vi "front_panel_v2.vi"() -> ()   [LabVIEW 2021]
uses:
  <vilib>/Platform/TimedLoop/XDataNode/timing_clust.ctl
  <vilib>/Platform/TimedLoop/XDataNode/nitl_modes.ctl
  <vilib>/Platform/TimedLoop/XDataNode/wakeup.ctl
  Global 1.vi
  <vilib>/platform/TimedLoop/XDataNode/XDataNode.xnode
  <vilib>/Platform/TimedLoop/XDataNode/XDNodeRunTimeDep.lvlib
panel:
  in  "Glove Address":string
  in  "Robotic Hand Address":string="192.168.4.93"
  out "Thumb 3":dbl
  out "Index Finger 2":dbl
  out "Middle Finger3":dbl
  out "Ring Finger 3":dbl
  out "Pinky Finger 2":dbl
  out "Simulation Connected":bool
  in  "Stop":bool
  out "Hand Status":bool
  out "Glove Status":bool
  in  "Stop Execution":bool
  in  "?":enum32{"Imitation", "Manual Control"}(tab)=enum."Manual Control"
  out "Glove Signal":dbl[](array[numeric])
  in  "Stop Imitation":bool
  out "Finger Positions From Glove":dbl[](graph)
  out "Finger Positions":T1(graph)
  in  "Stop Manual Control":bool
  out "Output From Knob":string
  in  "Pinky":dbl(slide) scale=0.0..-47.0
  in  "Ring Finger":dbl(slide) scale=0.0..-60.0
  in  "Index":dbl(slide) scale=0.0..-20.0
  in  "Middle Finger":dbl(slide)=85.0 scale=85.0..4.0
  in  "Thumb":dbl(slide)=90.0
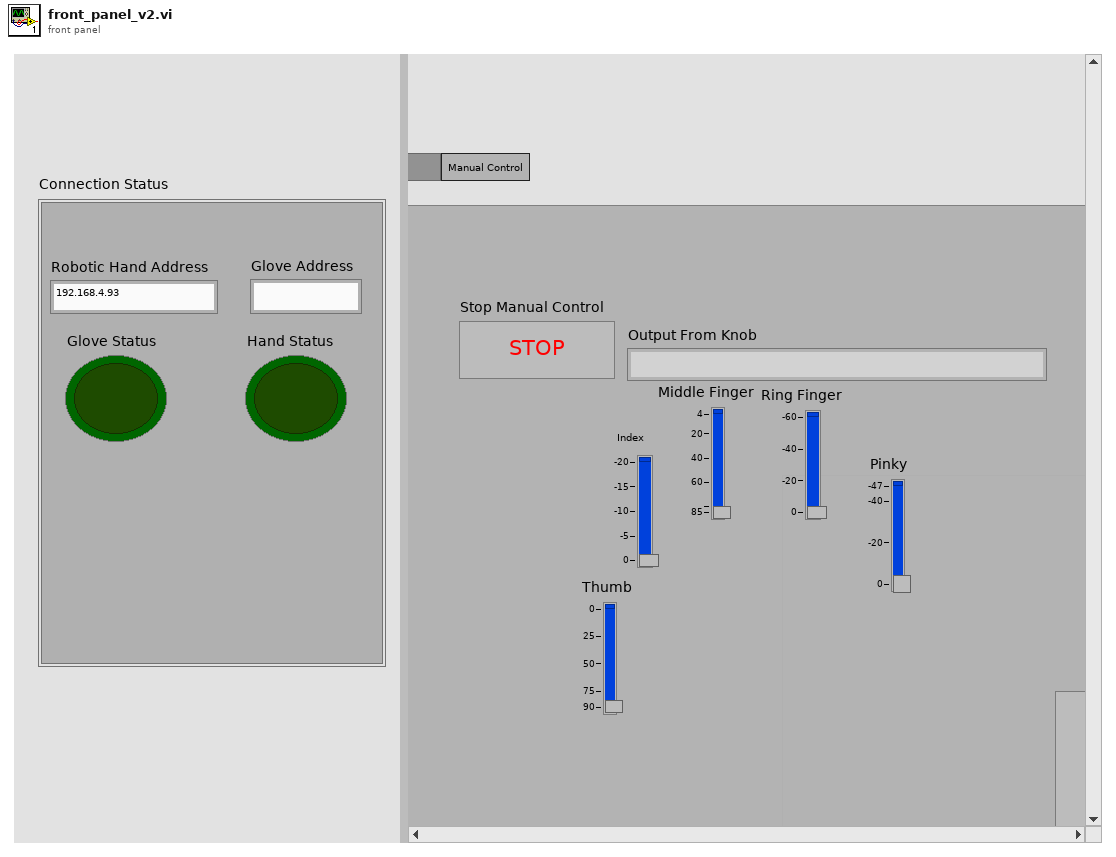
[diagram p1: front panel]
types:
  T1 = cluster{"[0]":dbl, "[1]":dbl, "[2]":dbl, "[3]":dbl, "[4]":dbl, "[5]":dbl, "[6]":dbl, "[7]":dbl, "[8]":dbl}
  T2 = cluster{"Clients":refnum<k5>[], "Listener":refnum<k5>}
  T3 = enum16{"Initialize", "Status Check", "Send Data", "Stop"}
  T4 = enum16{"Standard", "Buffered", "CRLF", "Immediate"}
  T5 = typedef "XDNodeRunTimeDep.lvlib/timing_clust.ctl" = cluster{"Expected End [f-1]":u64, "Actual End [f-1]":u64, "Finished Late? [f-1]":bool, "Expected End [i-1]":u64, "Actual End [i-1]":u64, "Finished Late? [i-1]":bool, "Expected Start [i]":u64, "Actual Start [i]":u64, "Expected Start [f]":u64, "Actual Start [f]":u64, "Source Name":string, "Structure Name":string, "Period":i64, "Deadline":i64, "Offset":i64, "Start":i64, "Priority":i32, "Timeout":i32, "Mode":T6, "Wakeup Reason":T7, "Error":errorcluster, "Source Type":string, "Secondary Source Type":string, "Global End Time":u64, "Global Start Time":u64, "Frame Duration":u64, "Iteration Duration":u64, "Assigned CPU":i32, "I/O Scan Engine Mode":u32}
  T6 = typedef "XDNodeRunTimeDep.lvlib/nitl_modes.ctl" = enum32{"No Change", "Process missed periods, maintain original phase", "Discard missed periods, maintain original phase", "Process missed periods, ignore original phase", "Discard missed periods, ignore original phase"}
  T7 = typedef "XDNodeRunTimeDep.lvlib/wakeup.ctl" = enum32{"Normal", "Aborted", "Asynchronous wakeup", "Timing source error", "Timed loop error", "Timeout"}
  T8 = cluster{"Glove output RT[0]":dbl, "Glove output RT[1]":dbl, "Glove output RT[2]":dbl, "Glove output RT[3]":dbl, "Glove output RT[4]":dbl, "Glove output RT[5]":dbl, "Glove output RT[6]":dbl, "Glove output RT[7]":dbl, "Glove output RT[8]":dbl}
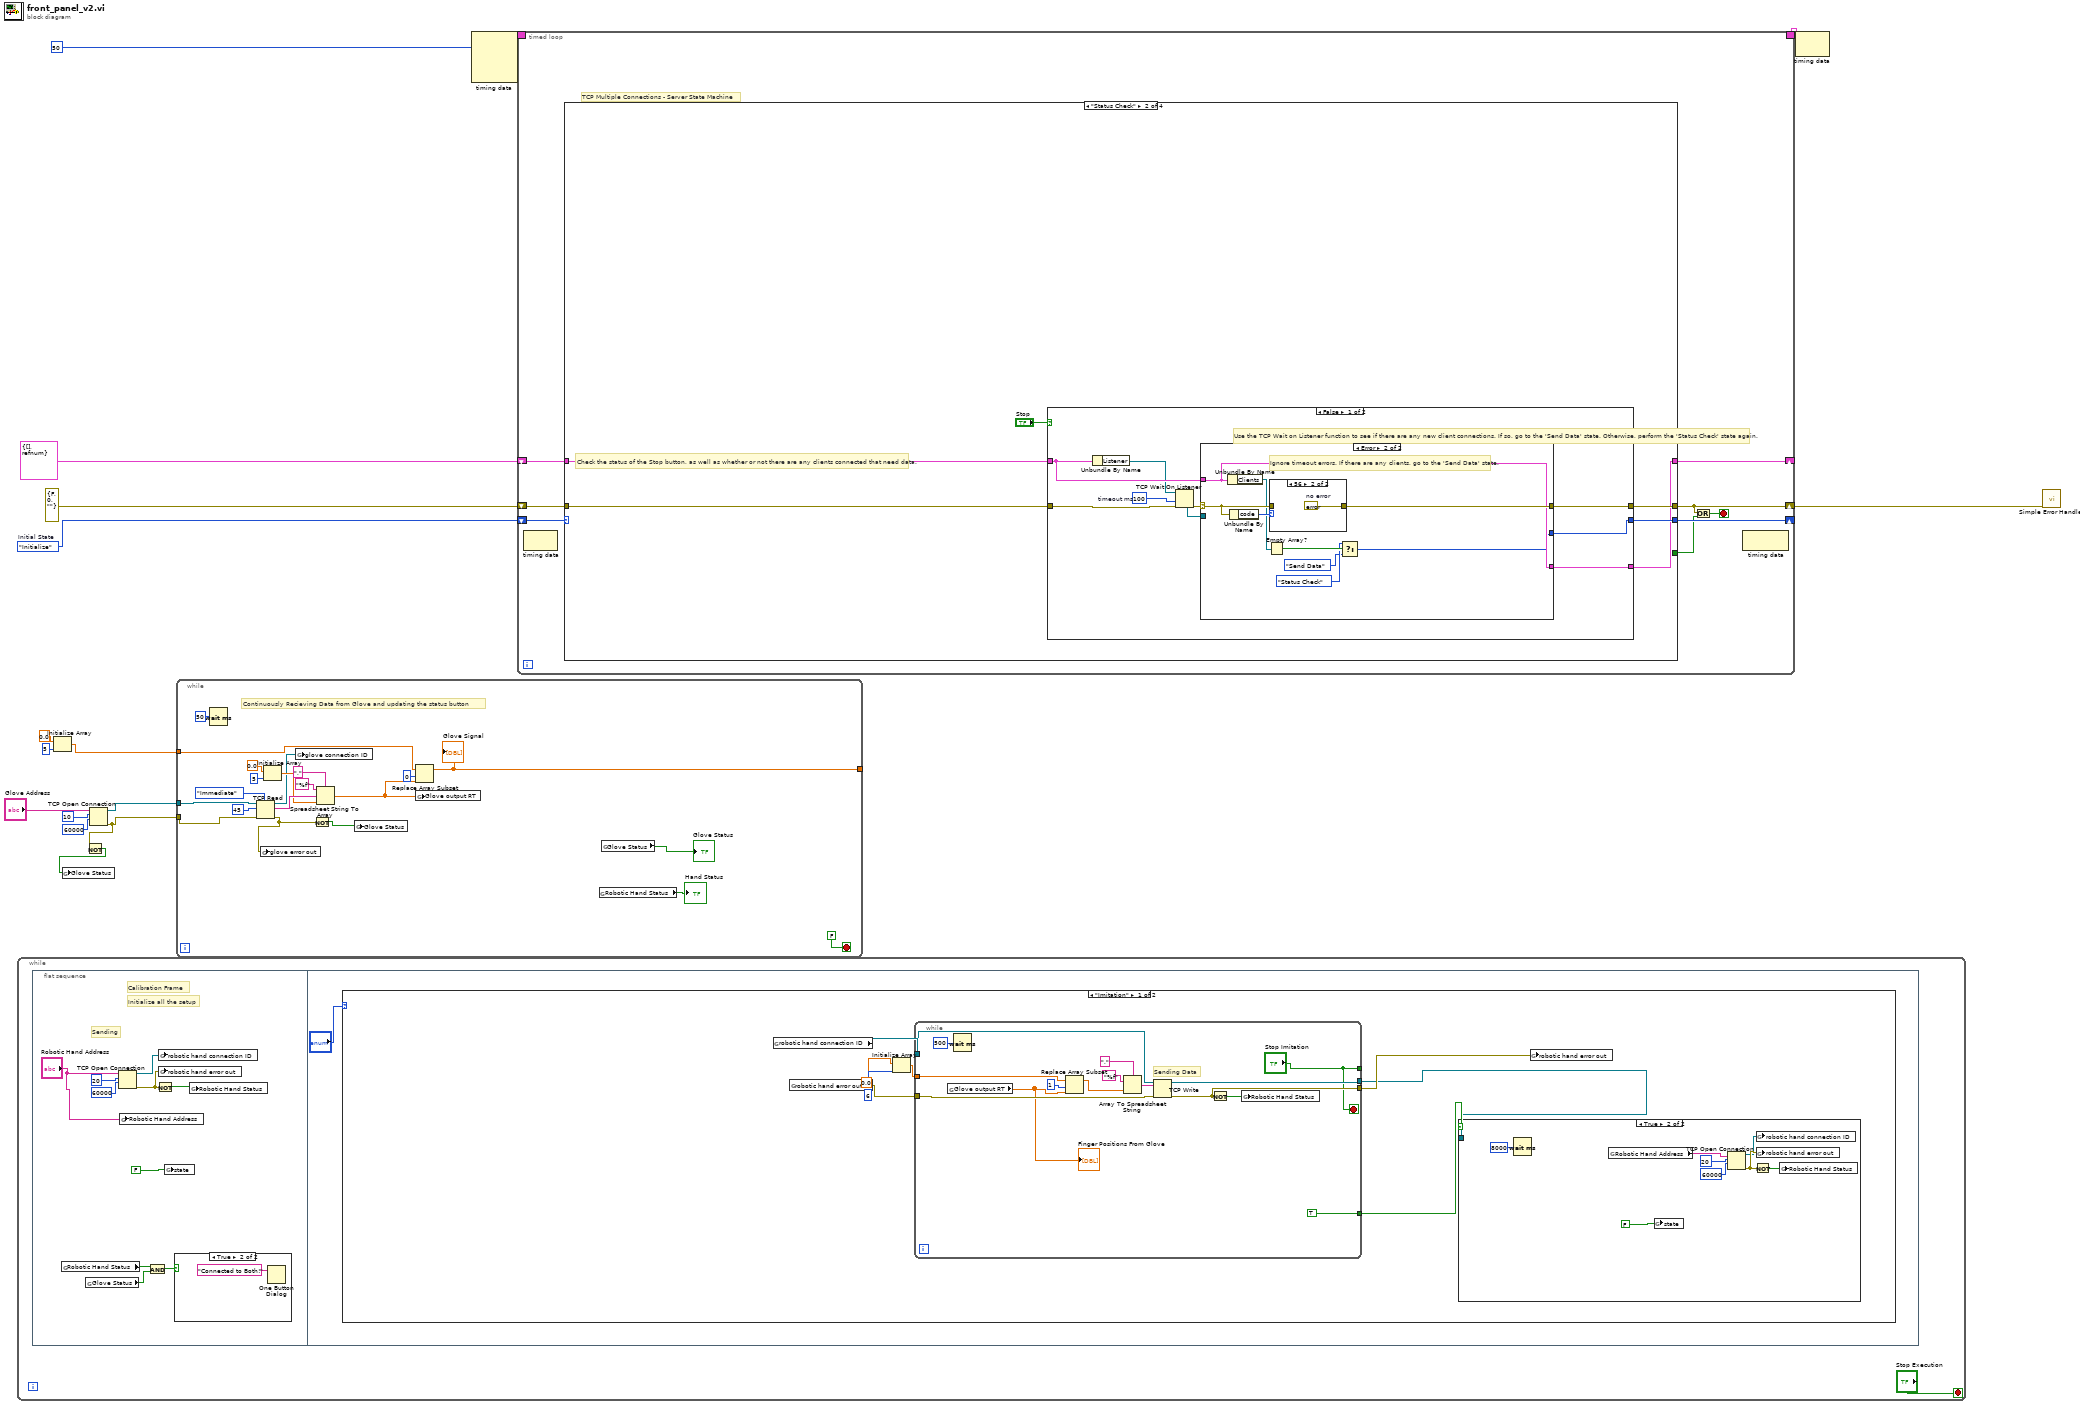
[diagram p0: block diagram]
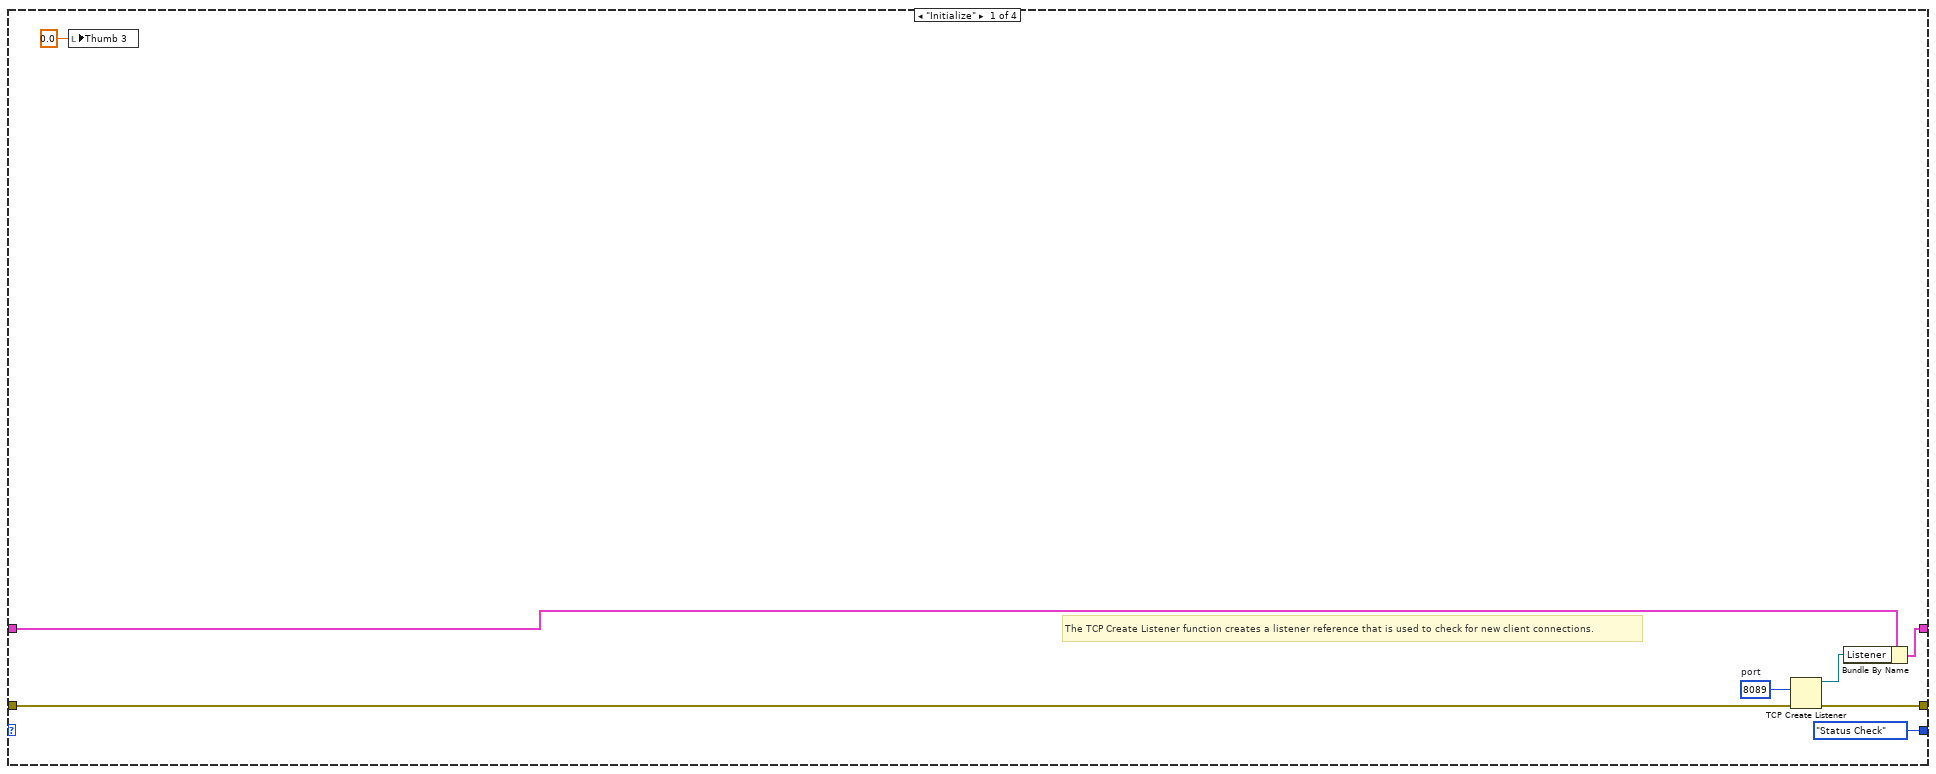
[diagram p2: hidden frame]
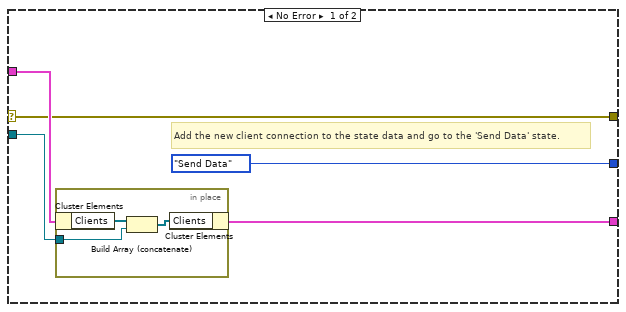
[diagram p3: hidden frame]
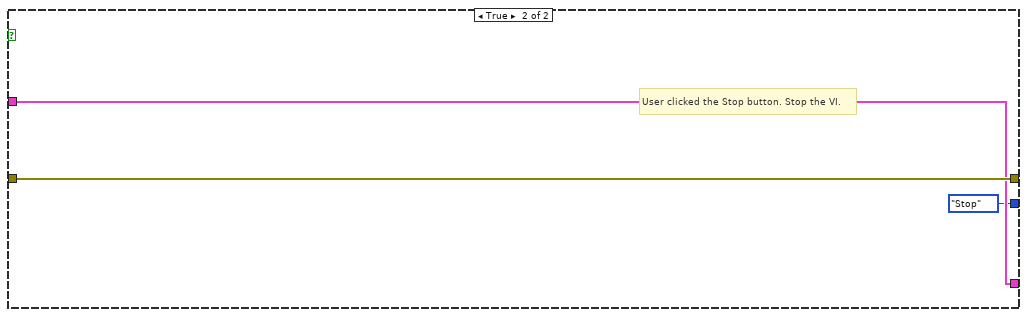
[diagram p5: hidden frame]
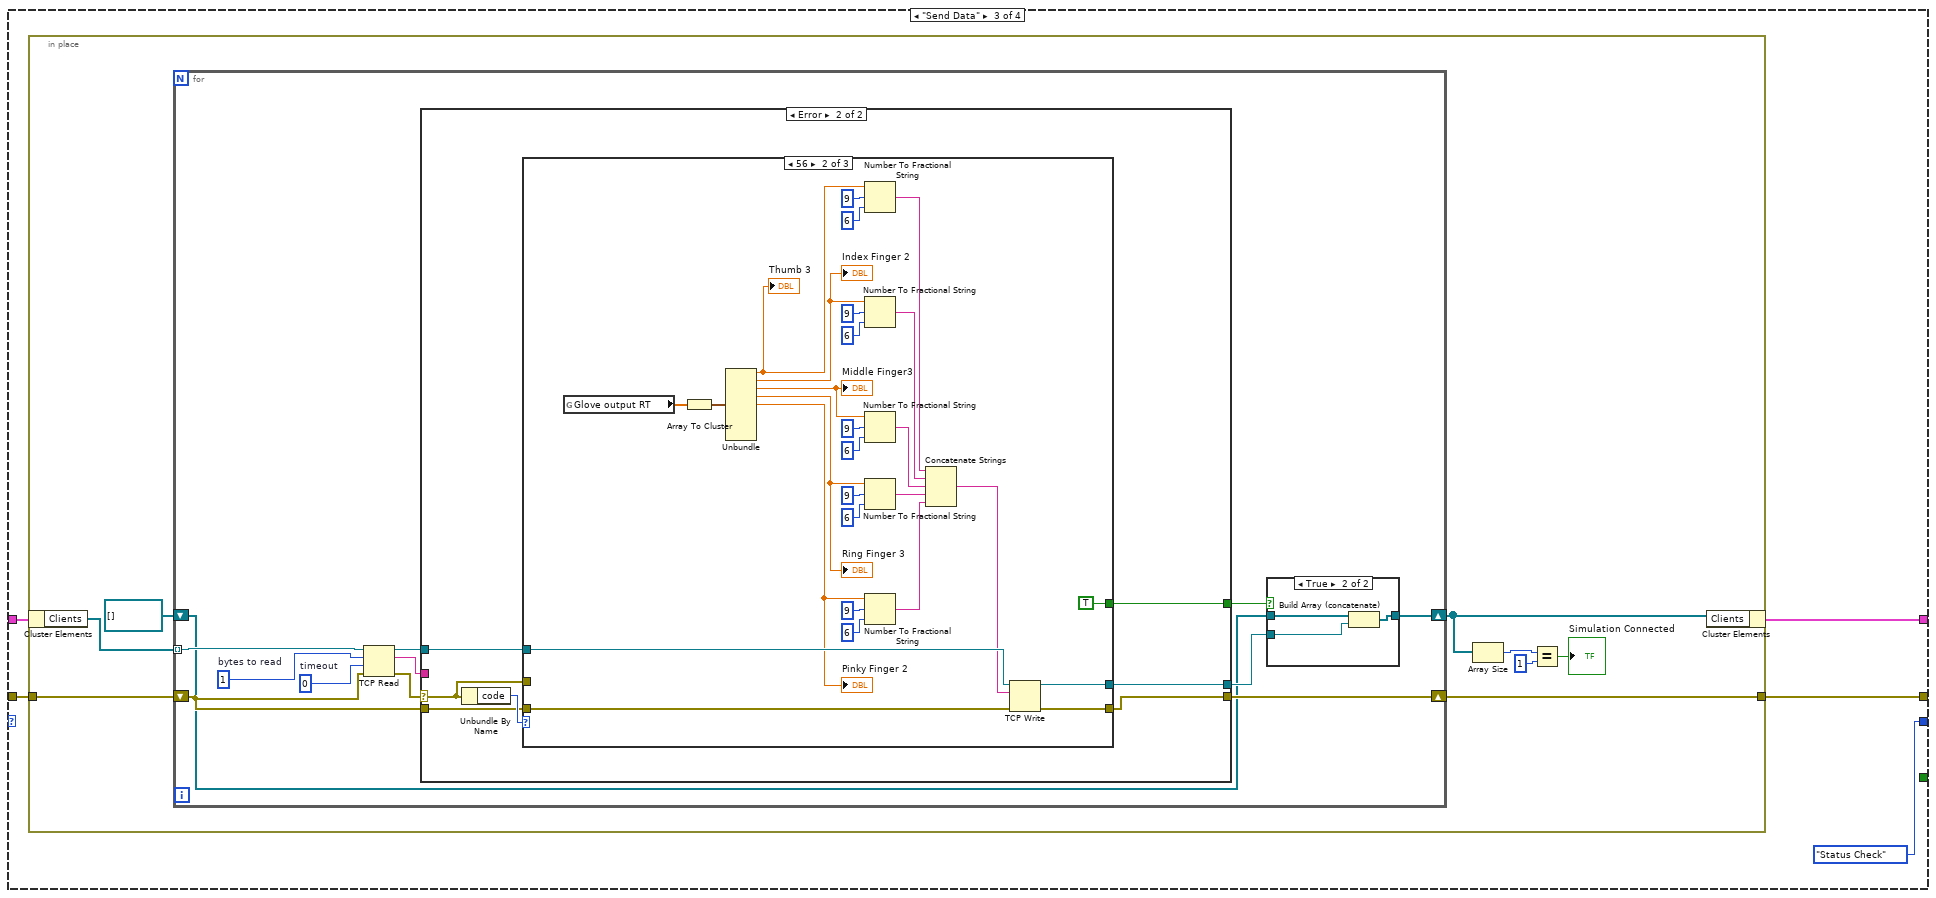
[diagram p6: hidden frame]
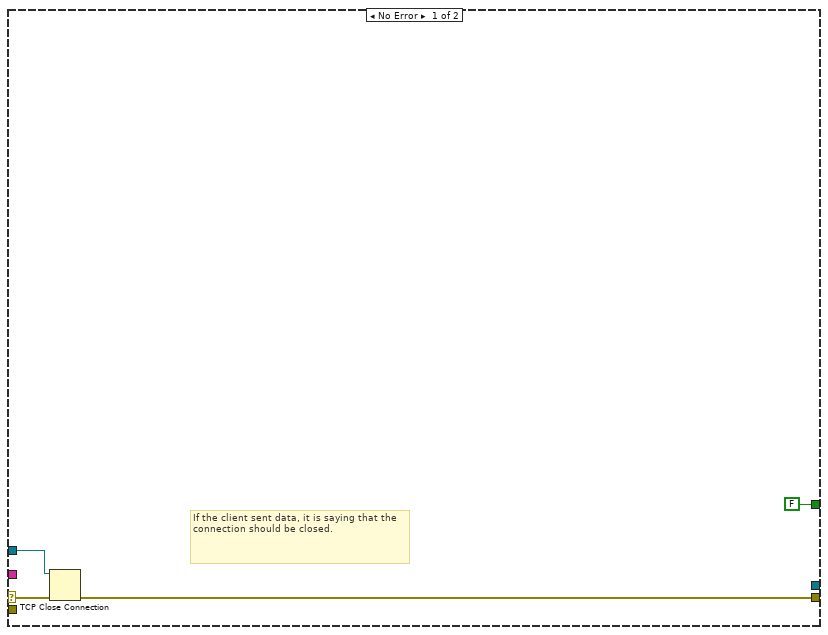
[diagram p8: hidden frame]
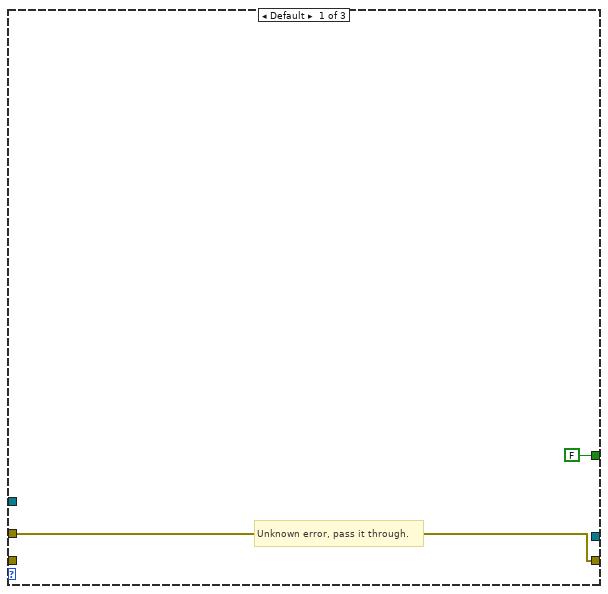
[diagram p9: hidden frame]
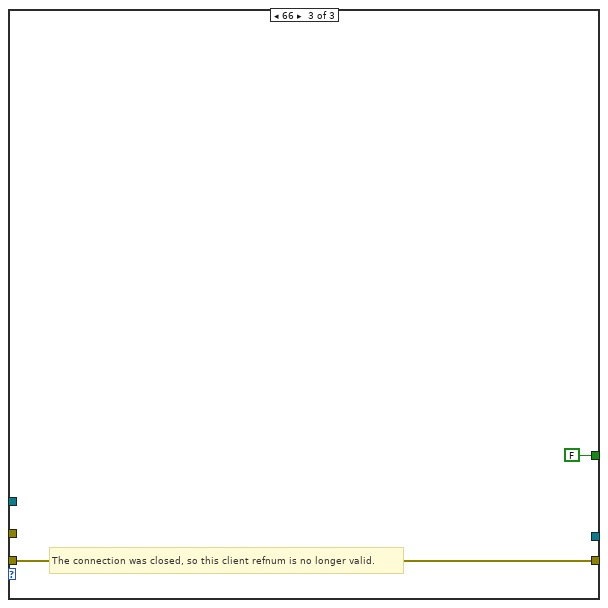
[diagram p10: hidden frame]
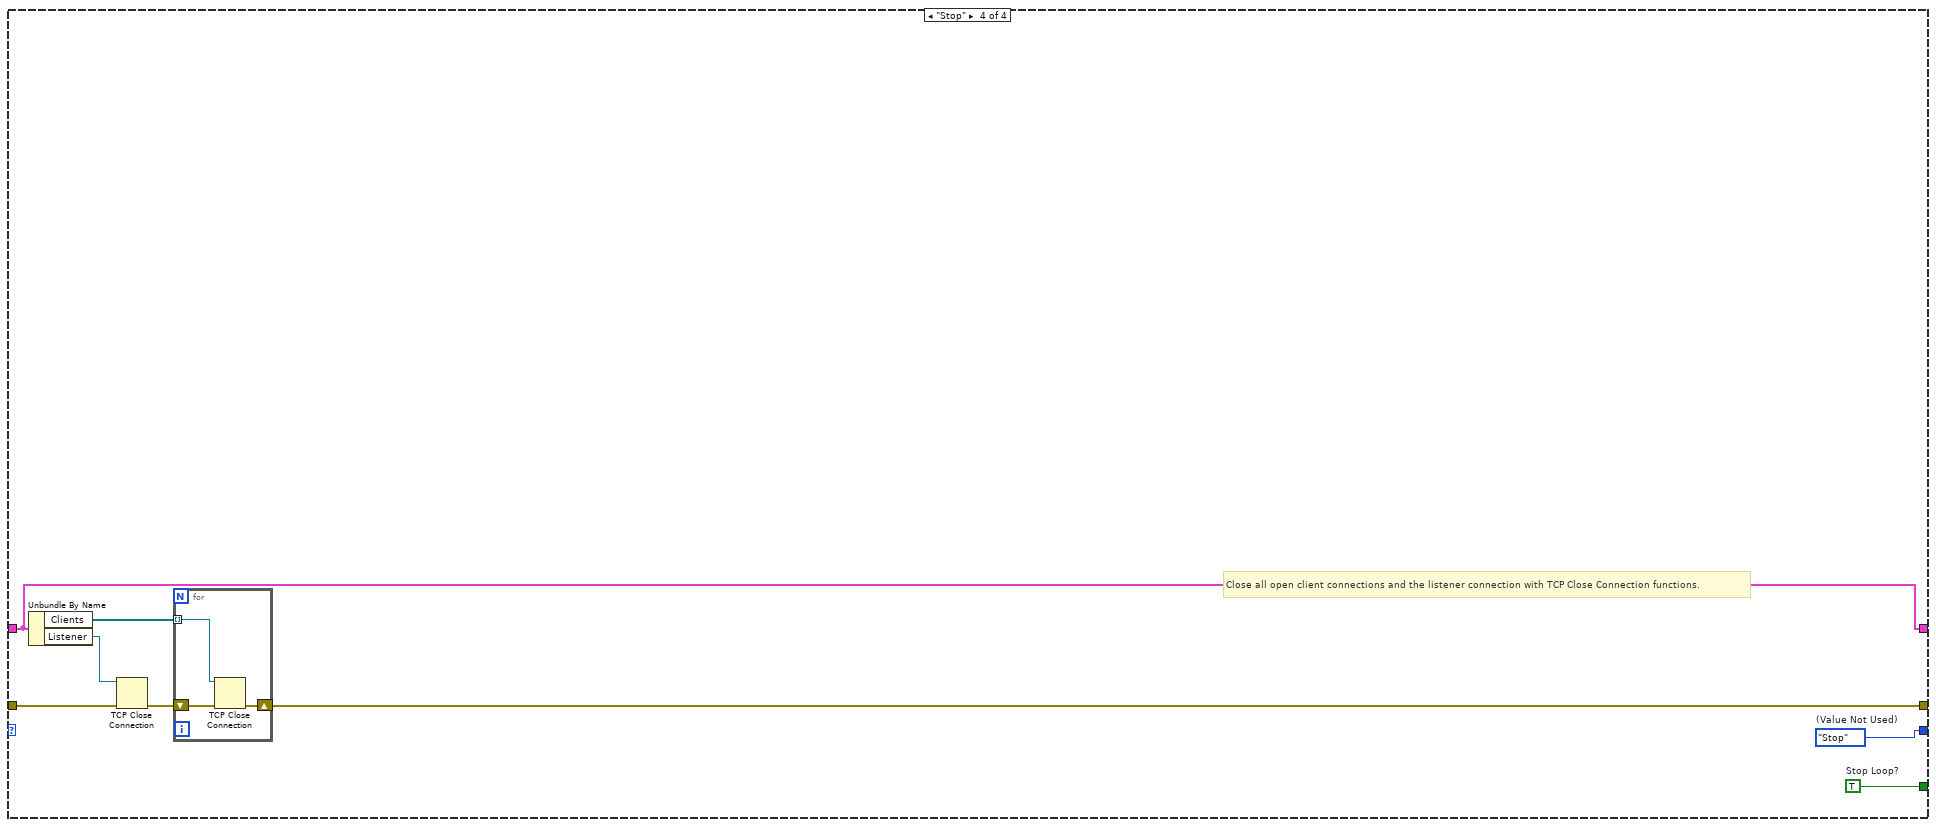
[diagram p11: hidden frame]
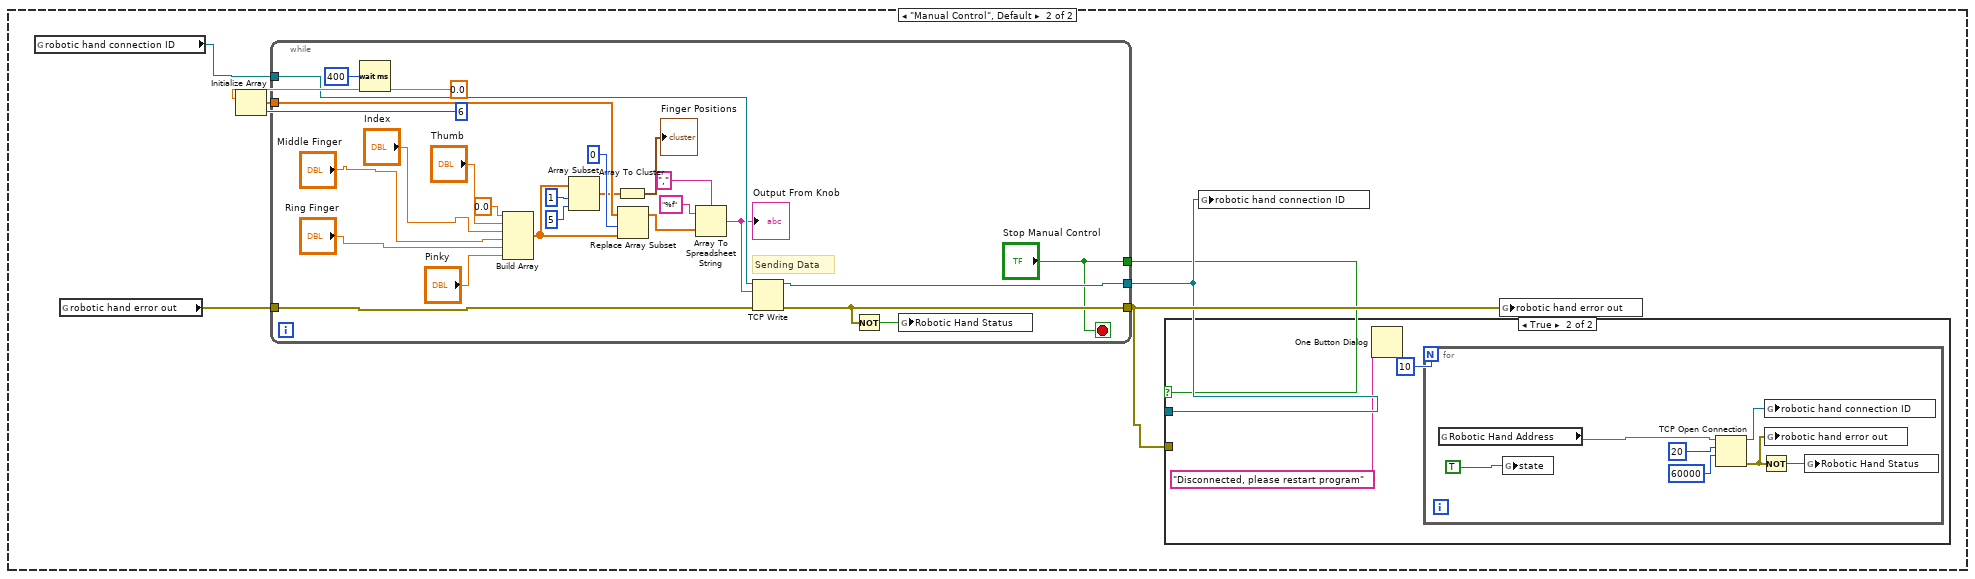
[diagram p14: hidden frame]
diagram:
  w16 = T3."Initialize"  # Initial State
  n1 = while {
    stop <- "Stop Execution" stop-if-true
    n2 = flat-sequence {
      frame #0 {
        # "Sending"
        # "Initialize all the setup"
        # "Calibration Frame"
        n3 = global read "Global 1.vi" "Robotic Hand Status"() -> (w25:bool)
        n4 = global read "Global 1.vi" "Glove Status"() -> (w26:bool)
        n5 = TCP Open Connection(address="Robotic Hand Address", remote port or service name=u16 20, timeout ms (60000)=60000) -> (connection ID=w22:refnum<k5>, error out=w23:errorcluster)  [unwired: 2 in]
        n6 = global write "Global 1.vi" "Robotic Hand Address"("Robotic Hand Address") -> ()
        n7 = And(x=w25, y=w26) -> (x .and. y?=w27:bool)
        n8 = Not(x=w23) -> (.not. x?=w24:bool)
        n9 = global write "Global 1.vi" "robotic hand connection ID"(w22) -> ()
        n10 = global write "Global 1.vi" "robotic hand error out"(w23) -> ()
        n11 = global write "Global 1.vi" "state"(FALSE ("Robotic Hand Status")) -> ()
        n12 = case shown="True" w27 {
          frame False {
          }
          frame True {
            n13 = One Button Dialog(message="Connected to Both!") -> ()  [unwired: 1 in, 1 out]
          }
        }
        n14 = global write "Global 1.vi" "Robotic Hand Status"(w24) -> ()
      }
      frame #1 {
        n15 = case shown="\"Imitation\"" "?" {
          frame "Imitation" {
            n16 = global read "Global 1.vi" "robotic hand connection ID"() -> (w35:refnum<k5>)
            n17 = global read "Global 1.vi" "robotic hand error out"() -> (w34:errorcluster)
            n18 = Initialize Array(0.0 ("element"), 6 ("dimension size")) -> (w36:dbl[])
            n19 = while {
              tunnel: [w60] -> w30
              tunnel: w35 -> [w59]
              tunnel: w34 -> [w57]
              tunnel: [w50] -> w33
              tunnel: w36 -> [w49]
              tunnel: ["Stop Imitation"] -> _
              tunnel: [TRUE] -> w31
              stop <- "Stop Imitation" stop-if-true
              # "Sending Data"
              n20 = global read "Global 1.vi" "Glove output RT"() -> (w46:dbl[])
              "Finger Positions From Glove" <- w46
              n21 = Wait (ms)(milliseconds to wait=u32 500) -> ()  [unwired: 1 out]
              n22 = Replace Array Subset(array=w49, new element=w46, index=1) -> (w54:dbl[])
              n23 = Array To Spreadsheet String(delimiter (Tab)=",", array=w54, 3:"%f" ("format string")) -> (spreadsheet string=w52:string)
              n24 = TCP Write(connection ID=w59, data in=w52, error in (no error)=w57) -> (connection ID out=w60:refnum<k5>, error out=w50:errorcluster)  [unwired: 1 in, 1 out]
              n25 = Not(x=w50) -> (.not. x?=w51:bool)
              n26 = global write "Global 1.vi" "Robotic Hand Status"(w51) -> ()
            }
            n27 = case shown="True" w31 {
              tunnel: w30 -> [_ _]
              frame False {
              }
              frame True {
                n28 = Wait (ms)(milliseconds to wait=u32 8000) -> ()  [unwired: 1 out]
                n29 = global read "Global 1.vi" "Robotic Hand Address"() -> (w39:string)
                n30 = global write "Global 1.vi" "state"(FALSE ("Robotic Hand Status")) -> ()
                n31 = TCP Open Connection(address=w39, remote port or service name=u16 20, timeout ms (60000)=60000) -> (connection ID=w43:refnum<k5>, error out=w44:errorcluster)  [unwired: 2 in]
                n32 = Not(x=w44) -> (.not. x?=w45:bool)
                n33 = global write "Global 1.vi" "robotic hand connection ID"(w43) -> ()
                n34 = global write "Global 1.vi" "robotic hand error out"(w44) -> ()
                n35 = global write "Global 1.vi" "Robotic Hand Status"(w45) -> ()
              }
            }
            n36 = global write "Global 1.vi" "robotic hand error out"(w33) -> ()
          }
          frame "Manual Control", Default {
            n37 = global read "Global 1.vi" "robotic hand connection ID"() -> (w65:refnum<k5>)
            n38 = global read "Global 1.vi" "robotic hand error out"() -> (w64:errorcluster)
            n39 = Initialize Array(0.0 ("element"), 6 ("dimension size")) -> (w66:dbl[])
            n40 = while {
              tunnel: [w101] -> w62
              tunnel: w65 -> [w100]
              tunnel: w64 -> [w98]
              tunnel: [w90] -> w63
              tunnel: w66 -> [w92]
              tunnel: ["Stop Manual Control"] -> w61
              stop <- "Stop Manual Control" stop-if-true
              # "Sending Data"
              n41 = Wait (ms)(milliseconds to wait=u32 400) -> ()  [unwired: 1 out]
              n42 = Build Array(0.0 ("element"), "Thumb", "Index", "Middle Finger", "Ring Finger", "Pinky") -> (w86:dbl[])
              n43 = Array Subset(array=w86, index=1, length=5) -> (w85:dbl[])
              n44 = Array To Cluster(array=w85) -> (cluster=→"Finger Positions":T1)
              n45 = Replace Array Subset(array=w92, new element=w86, index=0) -> (w95:dbl[])
              n46 = Array To Spreadsheet String(delimiter (Tab)=",", array=w95, 3:"%f" ("format string")) -> (spreadsheet string=w93:string)
              "Output From Knob" <- w93
              n47 = TCP Write(connection ID=w100, data in=w93, error in (no error)=w98) -> (connection ID out=w101:refnum<k5>, error out=w90:errorcluster)  [unwired: 1 in, 1 out]
              n48 = Not(x=w90) -> (.not. x?=w91:bool)
              n49 = global write "Global 1.vi" "Robotic Hand Status"(w91) -> ()
            }
            n50 = case shown="True" w61 {
              tunnel: w62 -> [_ _]
              tunnel: w63 -> [_ _]
              frame False {
              }
              frame True {
                n51 = One Button Dialog(message="Disconnected, please restart program") -> ()  [unwired: 1 in, 1 out]
                n52 = for {
                  N: 10 -> [_]
                  n53 = global read "Global 1.vi" "Robotic Hand Address"() -> (w72:string)
                  n54 = global write "Global 1.vi" "state"(TRUE ("Robotic Hand Status")) -> ()
                  n55 = TCP Open Connection(address=w72, remote port or service name=u16 20, timeout ms (60000)=60000) -> (connection ID=w75:refnum<k5>, error out=w76:errorcluster)  [unwired: 2 in]
                  n56 = Not(x=w76) -> (.not. x?=w77:bool)
                  n57 = global write "Global 1.vi" "robotic hand connection ID"(w75) -> ()
                  n58 = global write "Global 1.vi" "robotic hand error out"(w76) -> ()
                  n59 = global write "Global 1.vi" "Robotic Hand Status"(w77) -> ()
                }
              }
            }
            n60 = global write "Global 1.vi" "robotic hand connection ID"(w62) -> ()
            n61 = global write "Global 1.vi" "robotic hand error out"(w63) -> ()
          }
        }
      }
    }
  }
  n62 = Initialize Array(0.0 ("element"), 5 ("dimension size")) -> (w3:dbl[])
  n63 = TCP Open Connection(address="Glove Address", remote port or service name=u16 10, timeout ms (60000)=60000) -> (connection ID=w8:refnum<k5>, error out=w9:errorcluster)  [unwired: 2 in]
  n64 = Not(x=w9) -> (.not. x?=w12:bool)
  n65 = global write "Global 1.vi" "Glove Status"(w12) -> ()
  n66 = while {
    tunnel: w8 -> [w109]
    tunnel: w9 -> [w108]
    tunnel: w3 -> [w103]
    tunnel: [w102] -> _
    stop <- FALSE stop-if-true
    # "Continuously Recieving Data from Glove and updating the status button"
    n67 = Wait (ms)(milliseconds to wait=u32 50) -> ()  [unwired: 1 out]
    n68 = TCP Read(connection ID=w109, bytes to read=45, error in (no error)=w108, 7:T4."Immediate" ("mode (standard)")) -> (connection ID out=w110:refnum<k5>, data out=w116:string, error out=w106:errorcluster)  [unwired: 1 in]
    n69 = global write "Global 1.vi" "glove error out"(w106) -> ()
    n70 = Initialize Array(0.0 ("element"), 5 ("dimension size")) -> (w115:dbl[])
    n71 = global write "Global 1.vi" "glove connection ID"(w110) -> ()
    n72 = Not(x=w106) -> (.not. x?=w107:bool)
    n73 = Spreadsheet String To Array(delimiter (Tab)=",", format string="%f", spreadsheet string=w116, array type (2D Dbl)=w115) -> (array=w105:dbl[])
    n74 = global write "Global 1.vi" "Glove Status"(w107) -> ()
    n75 = Replace Array Subset(array=w103, new element=w105, index=0) -> (w102:dbl[])
    "Glove Signal" <- w102
    n76 = global write "Global 1.vi" "Glove output RT"(w105) -> ()
    n77 = global read "Global 1.vi" "Robotic Hand Status"() -> (→"Hand Status":bool)
    n78 = global read "Global 1.vi" "Glove Status"() -> (→"Glove Status":bool)
  }
  n79 = node-c288(i64 50 ("Period")) -> (w7:T5)  [unwired: 3 in]
  n80 = timed-loop {
    shift-right: [w129] -> _
    shift-left: w16 -> [w130]
    shift-right: [w127] -> _
    shift-left: T2 {"Clients"=[], "Listener"=refnum} ("Data") -> [w128]
    shift-right: [w123] -> w14
    shift-left: errorcluster {"status"=FALSE, "code"=0, "source"=""} ("error constant") -> [w126]
    timing: w7 -> [_]
    timing-out: [_] -> w6
    stop <- w124 stop-if-true
    # "TCP Multiple Connections - Server State Machine"
    n81 = node-c288() -> ()  [unwired: 1 in, 1 out]
    n82 = case shown="\"Status Check\"" w130 {
      tunnel: [T3."Status Check" ("States") w146 T3."Status Check" ("States") w250] -> w129
      tunnel: [_ _ _ w257] -> w125
      tunnel: w128 -> [w138 w142 w180 w256]
      tunnel: [w137 w141 w179 w256] -> w127
      tunnel: w126 -> [w140 w145 w182 w255]
      tunnel: [w139 w144 w181 w253] -> w123
      frame "Initialize" {
        w135 = u16 8089  # port
        # "The TCP Create Listener function creates a listener reference that is used to check for new client connections."
        n83 = local write "Thumb 3"(0.0 ("Current Data")) -> ()
        n84 = TCP Create Listener(8:w140, 10:w135) -> (0:w139:errorcluster, 3:w136:refnum<k5>)  [unwired: 4 out]
        n85 = Bundle By Name(cluster=w138, "Listener"=w136) -> (w137:T2)
      }
      frame "Status Check" {
        # "Check the status of the Stop button, as well as whether or not there are any clients connected that need data."
        n86 = case shown="False" "Stop" {
          tunnel: [w155 T3."Stop" ("States")] -> w146
          tunnel: w145 -> [w154 w177]
          tunnel: [w147 w177] -> w144
          tunnel: w142 -> [w150 w176]
          tunnel: [w149 w176] -> w141
          frame False {
            w153 = 100  # timeout ms
            # "Use the TCP Wait on Listener function to see if there are any new client connections. If so, go to the 'Send Data' state. Otherwise, perform the 'Status Check' state again."
            n87 = Unbundle By Name(w150) -> ("Listener"=w148:refnum<k5>)
            n88 = TCP Wait On Listener(8:w154, 9:w153, 11:w148) -> (0:w152:errorcluster, 4:w151:refnum<k5>)  [unwired: 4 out]
            n89 = case shown="Error" w152 {
              selector: w152 -> [w158 w172]
              tunnel: [T3."Send Data" ("States") w166] -> w155
              tunnel: w151 -> [w159 _]
              tunnel: w150 -> [w160 w169]
              tunnel: [w157 w169] -> w149
              tunnel: [w158 w170] -> w147
              frame No Error {
                # "Add the new client connection to the state data and go to the 'Send Data' state."
                n90 = in-place {
                  in-place-border: w159 -> [w161]
                  n91 = in-place-cluster #1(w160) -> ("Clients"=w163:refnum<k5>[])
                  n92 = Build Array (concatenate)(w163, w161) -> (w162:refnum<k5>[])
                  n93 = in-place-cluster #1("Clients"=w162) -> (w157:T2)
                }
              }
              frame Error {
                # "Ignore timeout errors. If there are any clients, go to the 'Send Data' state."
                n94 = Unbundle By Name(w169) -> ("Clients"=w168:refnum<k5>[])
                n95 = Unbundle By Name(w172) -> ("code"=w171:i32)
                n96 = Empty Array?(array=w168) -> (empty?=w167:bool)
                n97 = case shown="56" w171 {
                  tunnel: w172 -> [w173 _]
                  tunnel: [w173 w174] -> w170
                  frame Default {
                  }
                  frame 56 {
                    w174 = errorcluster {"status"=FALSE, "code"=0, "source"=""}  # no error
                  }
                }
                n98 = Select(t=T3."Status Check" ("States"), s=w167, f=T3."Send Data" ("States")) -> (s? t:f=w166:T3)
              }
            }
          }
          frame True {
            # "User clicked the Stop button. Stop the VI."
          }
        }
      }
      frame "Send Data" {
        n99 = in-place {
          in-place-border: w182 -> [w190]
          in-place-border: [w189] -> w181
          n100 = in-place-cluster #2(w180) -> ("Clients"=w188:refnum<k5>[])
          n101 = for {
            tunnel: w188 -> [w202] mode=indexing
            shift-right: [w194] -> w189
            shift-left: w190 -> [w193]
            shift-right: [w191] -> w187
            shift-left: refnum<k5>[] [] ("Array") -> [w192]
            w199 = 0  # timeout
            w200 = 1  # bytes to read
            n102 = TCP Read(connection ID=w202, bytes to read=w200, error in (no error)=w193, 9:w199) -> (connection ID out=w201:refnum<k5>, data out=w197:string, error out=w198:errorcluster)  [unwired: 1 out]
            n103 = case shown="Error" w198 {
              selector: w198 -> [w209 w216]
              tunnel: w201 -> [w210 w213]
              tunnel: w197 -> [_ _]
              tunnel: [_ w211] -> w196
              tunnel: [FALSE w212] -> w195
              tunnel: [w207 w215] -> w194
              tunnel: w193 -> [_ w214]
              frame No Error {
                # "If the client sent data, it is saying that the connection should be closed."
                # "If the client sent data, it is saying that the connection should be closed."
                n104 = TCP Close Connection(connection ID=w210, error in (no error)=w209) -> (error out=w207:errorcluster)  [unwired: 2 out]
              }
              frame Error {
                # "Ignore connection closed and timeout errors"
                n105 = Unbundle By Name(w216) -> ("code"=w217:i32)
                n106 = case shown="56" w217 {
                  tunnel: w216 -> [w219 _ _]
                  tunnel: [w219 w247 w249] -> w215
                  tunnel: w214 -> [_ w243 w249]
                  tunnel: w213 -> [_ w246 _]
                  tunnel: [FALSE TRUE FALSE] -> w212
                  tunnel: [_ w245 _] -> w211
                  frame Default {
                    # "Unknown error, pass it through."
                  }
                  frame 56 {
                    n107 = global read "Global 1.vi" "Glove output RT"() -> (w226:dbl[])
                    n108 = Array To Cluster(array=w226) -> (cluster=w225:T8)
                    n109 = Unbundle(w225) -> ("Glove output RT[0]"=w222:dbl, "Glove output RT[1]"=w223:dbl, "Glove output RT[2]"=w224:dbl, "Glove output RT[3]"=w221:dbl, "Glove output RT[4]"=w220:dbl)  [unwired: 4 out]
                    "Thumb 3" <- w222
                    "Index Finger 2" <- w223
                    "Middle Finger3" <- w224
                    "Ring Finger 3" <- w221
                    "Pinky Finger 2" <- w220
                    n110 = Number To Fractional String(number=w222, width (-)=i16 9, precision (6)=i16 6) -> (F-format string=w241:string)  [unwired: 1 in]
                    n111 = Number To Fractional String(number=w223, width (-)=i16 9, precision (6)=i16 6) -> (F-format string=w240:string)  [unwired: 1 in]
                    n112 = Number To Fractional String(number=w224, width (-)=i16 9, precision (6)=i16 6) -> (F-format string=w239:string)  [unwired: 1 in]
                    n113 = Number To Fractional String(number=w221, width (-)=i16 9, precision (6)=i16 6) -> (F-format string=w238:string)  [unwired: 1 in]
                    n114 = Number To Fractional String(number=w220, width (-)=i16 9, precision (6)=i16 6) -> (F-format string=w237:string)  [unwired: 1 in]
                    n115 = Concatenate Strings(w241, w240, w239, w238, w237) -> (w242:string)
                    n116 = TCP Write(connection ID=w246, data in=w242, error in (no error)=w243) -> (connection ID out=w245:refnum<k5>, error out=w247:errorcluster)  [unwired: 2 out]
                  }
                  frame 66 {
                    # "The connection was closed, so this client refnum is no longer valid."
                  }
                }
              }
            }
            n117 = case shown="True" w195 {
              tunnel: w192 -> [w203 w205]
              tunnel: w196 -> [_ w204]
              tunnel: [w203 w206] -> w191
              frame False {
              }
              frame True {
                n118 = Build Array (concatenate)(w205, w204) -> (w206:refnum<k5>[])
              }
            }
          }
          n119 = Array Size(array=w187) -> (size(s)=w185:i32)
          n120 = Equal?(x=w185, y=1) -> (x = y?=→"Simulation Connected":bool)
          n121 = in-place-cluster #2("Clients"=w187) -> (w179:T2)
        }
      }
      frame "Stop" {
        w250 = T3."Stop"  # (Value Not Used)
        w257 = TRUE  # Stop Loop?
        # "Close all open client connections and the listener connection with TCP Close Connection functions."
        n122 = Unbundle By Name(w256) -> ("Clients"=w254:refnum<k5>[], "Listener"=w251:refnum<k5>)
        n123 = TCP Close Connection(connection ID=w251, error in (no error)=w255) -> (error out=w252:errorcluster)  [unwired: 1 in, 1 out]
        n124 = for {
          shift-right: [w259] -> w253
          shift-left: w252 -> [w260]
          tunnel: w254 -> [w258] mode=indexing
          n125 = TCP Close Connection(connection ID=w258, error in (no error)=w260) -> (error out=w259:errorcluster)  [unwired: 1 in, 1 out]
        }
      }
    }
    n126 = Or(x=w123, y=w125) -> (x .or. y?=w124:bool)
    n127 = node-c288() -> ()  [unwired: 1 in, 1 out]
  }
  n128 = node-c288(w6) -> ()  [unwired: 1 out]
  n129 = call <vilib>:"Simple Error Handler.vi"("error in (no error)"=w14) -> ()  [unwired: 4 in, 5 out]
